vi "RealSense_HelloWorld_PointCloud.vi"() -> ()   [LabVIEW 2017]
doc: "Simple Demo showing how to connect a RealSense Camera to stream COLOR and DEPTH from the stereo camera of a D4xx series camera."
uses:
  <vilib>/Utility/miscctls.llb/LV3DPointTypeDef.ctl
  <vilib>/Utility/miscctls.llb/LVRGBAColorTypeDef.ctl
  <vilib>/picture/3D Picture Control/Object/Create Object (name).vi
  libRealSense3.lvlib
  <vilib>/picture/3D Picture Control/NI_3D Picture Control.lvlib
panel:
  in  "Color format":enum16{"Monochrome", "RGB internal (RGB)"}(ring)=enum."RGB internal (RGB)"
  in  "Display tab":T1(tab)
  out "Stream selection":u16(ring) items=["Depth + Left Color", "Unrectified L + R", "Rectified L + R", "Depth Only", "RGB ext. Only", "Depth + L Monochrome"]
  out "Found \nRealSense":bool=TRUE
  out "height":i32=720
  out "width":i32=1280
  out "init results":T2={"camera name"="Intel RealSense D415", "camera S/N"="725112060291", "F/W"="05.12.01.00", "Sensor name"="Stereo Module", "api_version"=23201, "rscontext"=2279652045952, "device_list"=2279390748064, "device count"=1, "Dev out"=2279652602464, "sensor_list"=2279759543328, "sensor count"=2, "Sensor out"=2279397784752}
  in  "Select Resolution":u16(ring)=29 items=["256 x 144 @90fps", "424 x 240 @6fps", "424 x 240 @15fps", "424 x 240 @30fps", "424 x 240 @60fps", "424 x 240 @90fps", "480 x 270 @6fps", "480 x 270 @15fps", "480 x 270 @30fps", "480 x 270 @60fps", "480 x 270 @90fps", "640 x 360 @6fps", "640 x 360 @15fps", "640 x 360 @30fps", "640 x 360 @60fps", "640 x 360 @90fps", "640 x 480 @6fps", "640 x 480 @15fps", "640 x 480 @30fps", "640 x 480 @60fps", "640 x 480 @90fps", "848 x 100 @100fps", "848 x 480 @6fps", "848 x 480 @15fps", "848 x 480 @30fps", "848 x 480 @60fps", "848 x 480 @90fps", "1280 x 720 @6fps", "1280 x 720 @15fps", "1280 x 720 @30fps"]
  in  "Sensor index":i32
  in  "Device index":i32
  out "L-R Baseline, mm":sgl=-54.83181
  out "fy":sgl=952.6064 format="%#_5g"
  out "fx":sgl=952.6064 format="%#_5g"
  out "ppy":sgl=370.69974 format="%#_5g"
  out "ppx":sgl=634.5728 format="%#_5g"
  in  "Exposure,us":sgl=33000.0
  in  "Autoexposure":bool=TRUE
  in  "Depth Presets":T3(ring)=enum."Face2"
  in  "Color Presets":T4(ring)=enum."DS410 (DS5a) 4"
  in  "Laser on/off":bool=TRUE
  in  "Gain(16-248)":sgl=16.0 min=16 max=248
  in  "Update Presets":bool
  in  "Laser \nPower (mW)":dbl(slide)=155.72448 min=0.0 max=360.0 scale=0.36..360.0
  in  "Range Scale":enum16{"200m", "100m", "60m", "6m", "2m", "1m"}(ring)=enum."6m"
  out "RGB image":picture
  out "Depth map":sgl[][](graph)
  out "3D Picture":refnum<vi>(3d-picture)
  out "init error":string="\rNo Error\rNo Error\rNo Error\rNo Error\rNo Error\rNo Error\rNo Error\r\rNo Error\rNo Error"
  out "Capture2 error":string="No Error"
  out "Start Error":string="No Error\rNo Error\rNo Error"
  out "Config error":string="No Error\rNo Error"
  out "Capture1 Error":string="No Error"
  out "Close Error":string="No Error\rNo Error\rNo Error\rNo Error"
  out "release frame error":string="No Error"
  out "iteration":i32=187
  in  "stop":bool=TRUE
  # "RealSense Hello World: PointCloud"
  # "This demo shows how to connect a RealSense D415 (not 435) Depth Camera, and display the textured PointCloud."
  # "Note; When you change Depth Preset you need to stop and restart for the HDAD settings to take effect.\n\nTry the Color preset called \"Remove IR2\". It will remove the laser projector from the RGB 1280x720 image."
  # "INTRINSICS & EXTRINSICS"
  # "SELECT THE RESOLUTION"
  # "Recommendation:\nFor D435: 848x480, D415: 1280x720"
  # "DEPTH MAP"
  # "COLOR"
  # "Changes Color scale for Depth Map."
  # "20-1660000"
  # "3D POINTCLOUD"
  # "Rotate: Drag image\nMove X-Y: HOLD DOWN CTRL while dragging.\nZoom: SHIFT while dragging."
  # "ERRORS"
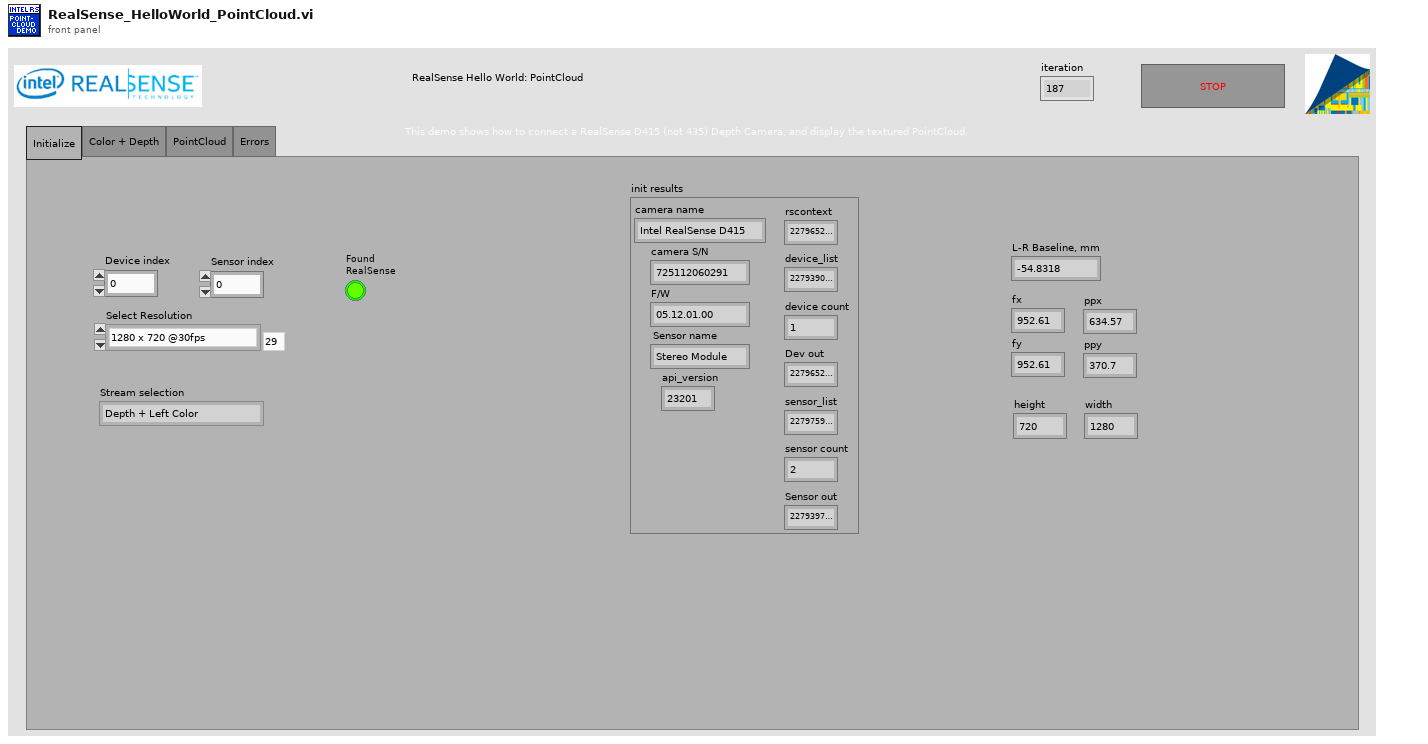
[diagram p1: front panel]
types:
  T1 = enum32{"Initialize", "Color + Depth", "PointCloud", "Errors"}
  T2 = cluster{"camera name":string, "camera S/N":string, "F/W":string, "Sensor name":string, "api_version":i32, "rscontext":u64, "device_list":u64, "device count":i32, "Dev out":u64, "sensor_list":u64, "sensor count":i32, "Sensor out":u64}
  T3 = enum16{"Custom", "Original", "New Depth 1", "New Depth 2", "Depth Active 1", "Active 3D Scan", "Active Short A", "Active Short C", "Face", "Face2", "Best Box", "High Density", "Medium Density", "High Accuracy", "Hand", "Short Range", "Flat wall", "Load .JSON", "Load .JSON2"}
  T4 = enum16{"Custom", "RS400 (DS5p)", "RS400 (DS5p) 2", "RS400 (DS5p) 3", "RS400 (DS5p) 4", "RS400 (DS5p) 5", "RS410 (DS5a)", "RS410 (DS5a) 2", "DS410 (DS5a) 3", "DS410 (DS5a) 4", "DS410+IR", "DS5LR", "DS5LR-2", "DS5LR no pattern", "RS410 Remove IR", "RS410 Remove IR 2", "DS5micro", "D435"}
  T5 = cluster{"width":i32, "height":i32, "fps":i32, "Profile":u64, "ppx":sgl, "ppy":sgl, "fx":sgl, "fy":sgl, "model":u32}
  T6 = enum16{"Overall", "Per Primitive", "Per Vertex", "Binding Off"}
  T7 = enum16{"Points", "Lines", "Line Strip", "Line Loop", "Triangles", "Triangle Strip", "Triangle Fan", "Quads", "Quad Strip", "Polygon"}
  T8 = enum16{"Depth", "Color (ext.)", "Color (left) ", "IR Left", "IR Right", "IR Left (Y16)", "IR Right (Y16)"}
  T9 = cluster{"R":dbl, "G":dbl, "B":dbl, "Alpha":dbl}[]
  T10 = typedef "LVRGBAColorTypeDef.ctl" = cluster{"Red":sgl, "Green":sgl, "Blue":sgl, "Alpha":sgl}
  T11 = typedef "LV3DPointTypeDef.ctl" = cluster{"X":sgl, "Y":sgl, "Z":sgl}
  T12 = cluster{"Alpha":sgl, "Blue":sgl, "Green":sgl, "Red":sgl}
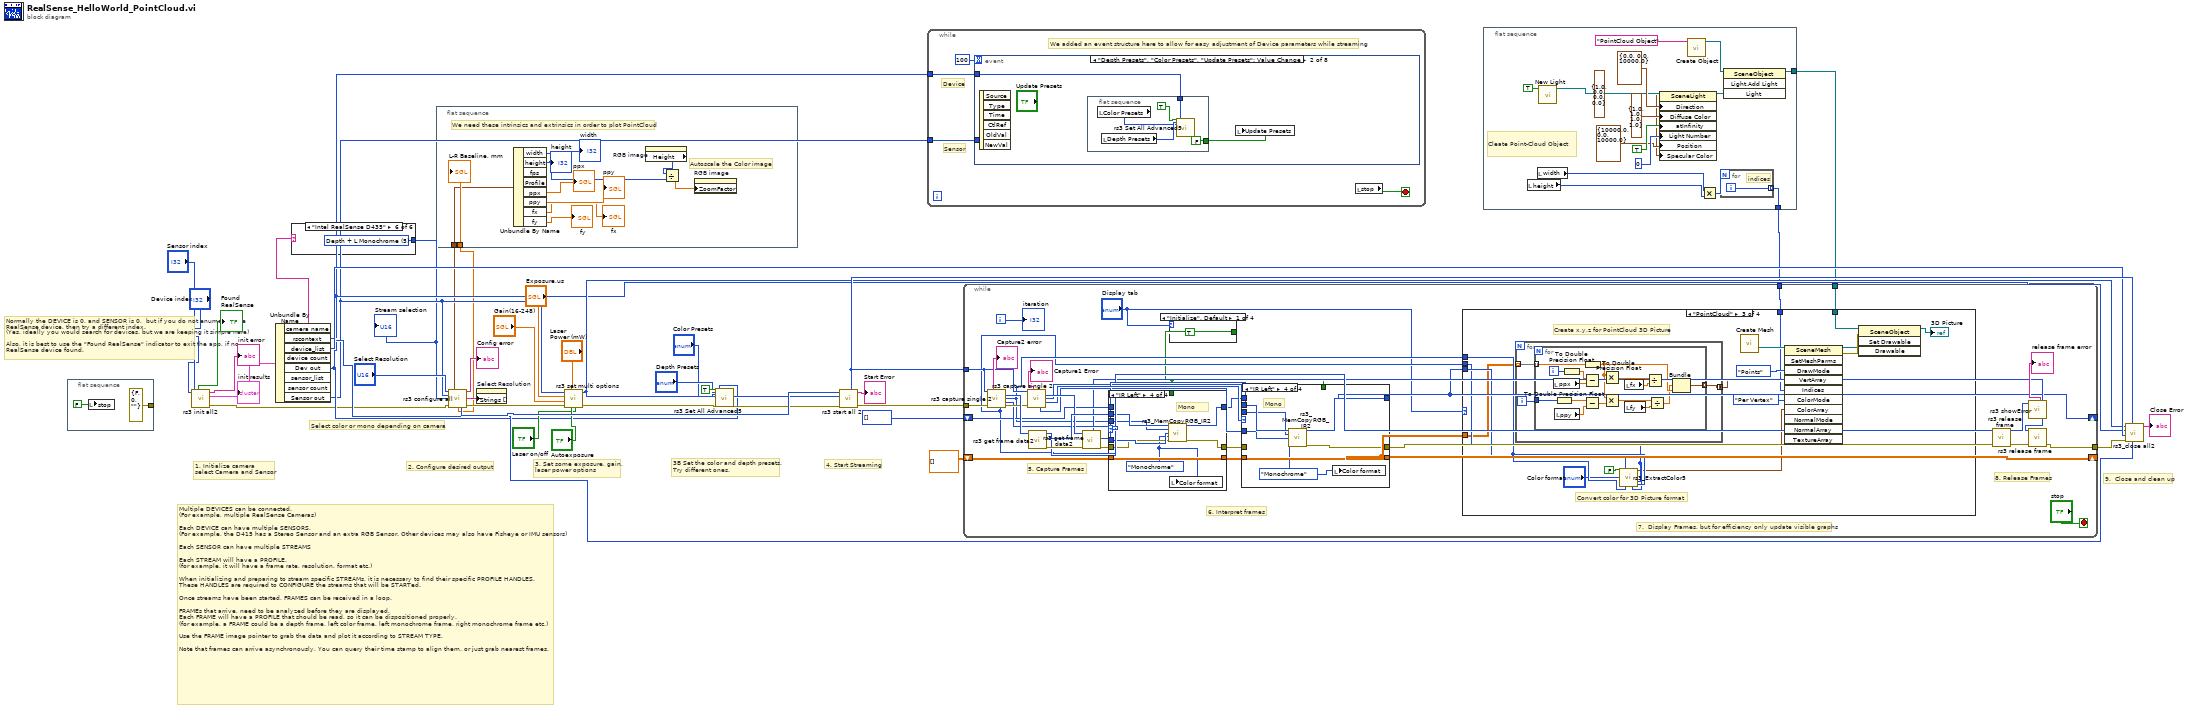
[diagram p0: block diagram]
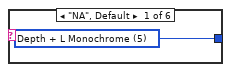
[diagram p2: hidden frame]
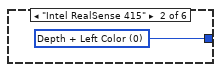
[diagram p3: hidden frame]
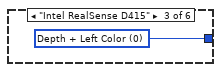
[diagram p4: hidden frame]
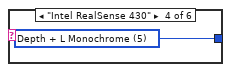
[diagram p5: hidden frame]
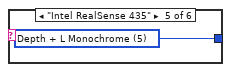
[diagram p6: hidden frame]
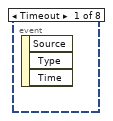
[diagram p7: hidden frame]
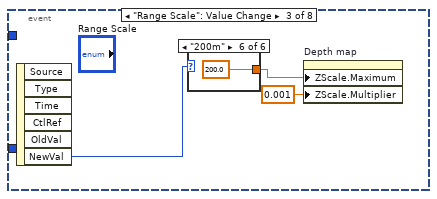
[diagram p8: hidden frame]
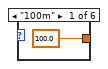
[diagram p9: hidden frame]
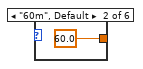
[diagram p10: hidden frame]
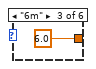
[diagram p11: hidden frame]
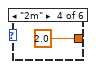
[diagram p12: hidden frame]
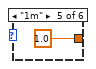
[diagram p13: hidden frame]
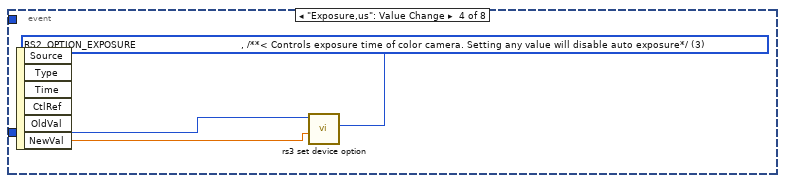
[diagram p14: hidden frame]
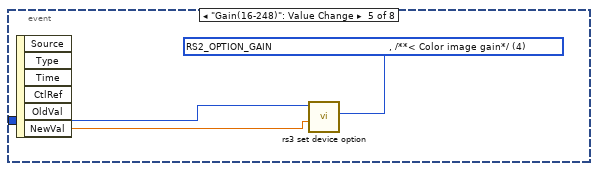
[diagram p15: hidden frame]
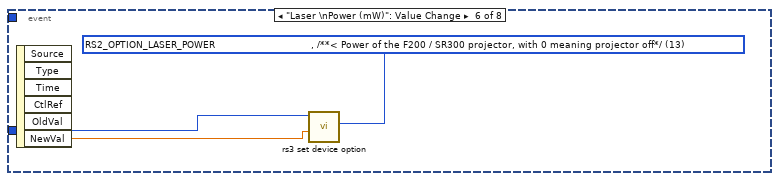
[diagram p16: hidden frame]
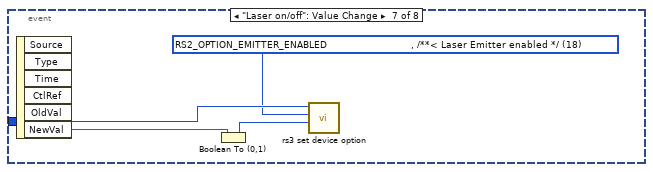
[diagram p17: hidden frame]
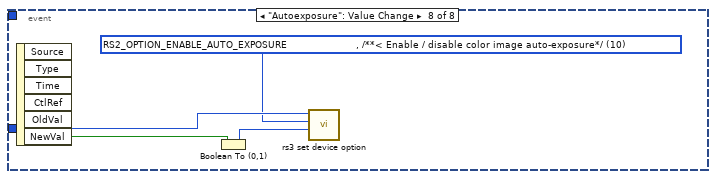
[diagram p18: hidden frame]
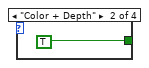
[diagram p19: hidden frame]
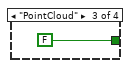
[diagram p20: hidden frame]
diagram:
  # "3B Set the color and depth presets.\nTry different ones."
  # "Select color or mono depending on camera"
  # "Normally the DEVICE is 0, and SENSOR is 0,  but if you do not enumerate the RealSense device, then try a different index.\n(Yes, ideally you would search for devices, but we are keeping it simple here)\n\nAlso, it is best to use the \"Found RealSense\" indicator to exit the app, if no RealSense device found."
  # "Multiple DEVICES can be connected. \n(For example, multiple RealSense Cameras)\n\nEach DEVICE can have multiple SENSORS. \n(For example, the D415 has a Stereo Sensor and an extra RGB Sensor. Other devices may also have Fisheye or IMU sensors) \n\nEach SENSOR can have multiple STREAMS\n\nEach STREAM will have a PROFILE. \n(for example, it will have a frame rate, resolution, format etc.)\n\nWhen initializing and preparing to stream specific STREAMs, it is necessary to find their specific PROFILE HANDLES.\nThese HANDLES are required to CONFIGURE the streams that will be STARTed. \n\nOnce streams have been started, FRAMES can be received in a loop. \n \nFRAMEs that arrive, need to be analyzed before they are displayed. \nEach FRAME will have a PROFILE that should be read, so it can be dispositioned properly.\n(for example, a FRAME could be a depth frame, left color frame, left monochrome frame, right monochrome frame etc.)\n\nUse the FRAME image pointer to grab the data and plot it according to STREAM TYPE.\n\nNote that frames can arrive asynchronously. You can query their time stamp to align them, or just grab nearest frames."
  # "9.  Close and clean up"
  # "4. Start Streaming"
  # "3. Set some exposure, gain, \nlaser power options"
  # "2. Configure desired output"
  # "1. Initialize camera\nselect Camera and Sensor"
  n1 = flat-sequence {
    tunnel: [errorcluster {"status"=FALSE, "code"=0, "source"=""} ("error in")] -> _
    frame #0 {
      n2 = local write "stop"(FALSE ("stop")) -> ()
    }
  }
  n3 = call "rs3 init all2.vi"("Select Device"="Device index", "Select Sensor"="Sensor index") -> ("error out"=w3:errorcluster, "init results"=w8:T2, "init error"=→"init error":string, "Found RealSense"=→"Found \nRealSense":bool)  [unwired: 3 in, 3 out]
  "init results" <- w8
  n4 = Unbundle By Name(w8) -> ("camera name"=w2:string, "rscontext"=w33:u64, "device_list"=w34:u64, "Dev out"=w16:u64, "Sensor out"=w15:u64)  [unwired: 3 out]
  n5 = case shown="\"Intel RealSense D435\"" w2 {
    tunnel: [w42 w43 w44 w45 w46 w47] -> w1
    frame "NA", Default {
      w42 = u16 5 items=["Depth + Left Color", "Unrectified L + R", "Rectified L + R", "Depth Only", "RGB ext. Only", "Depth + L Monochrome"] ("Stream selection")
    }
    frame "Intel RealSense 415" {
      w43 = u16 0 items=["Depth + Left Color", "Unrectified L + R", "Rectified L + R", "Depth Only", "RGB ext. Only", "Depth + L Monochrome"] ("Stream selection")
    }
    frame "Intel RealSense D415" {
      w44 = u16 0 items=["Depth + Left Color", "Unrectified L + R", "Rectified L + R", "Depth Only", "RGB ext. Only", "Depth + L Monochrome"] ("Stream selection")
    }
    frame "Intel RealSense 430" {
      w45 = u16 5 items=["Depth + Left Color", "Unrectified L + R", "Rectified L + R", "Depth Only", "RGB ext. Only", "Depth + L Monochrome"] ("Stream selection")
    }
    frame "Intel RealSense 435" {
      w46 = u16 5 items=["Depth + Left Color", "Unrectified L + R", "Rectified L + R", "Depth Only", "RGB ext. Only", "Depth + L Monochrome"] ("Stream selection")
    }
    frame "Intel RealSense D435" {
      w47 = u16 5 items=["Depth + Left Color", "Unrectified L + R", "Rectified L + R", "Depth Only", "RGB ext. Only", "Depth + L Monochrome"] ("Stream selection")
    }
  }
  "Stream selection" <- w1
  n6 = flat-sequence {
    tunnel: w13 -> [w57]
    tunnel: w12 -> [w56]
    frame #0 {
      # "Autoscale the Color image"
      # "We need these intrinsics and extrinsics in order to plot PointCloud"
      n7 = Unbundle By Name(w56) -> ("width"=→"width":i32, "height"=w54:i32, "ppx"=→"ppx":sgl, "ppy"=→"ppy":sgl, "fx"=→"fx":sgl, "fy"=→"fy":sgl)  [unwired: 2 out]
      "height" <- w54
      n8 = property on="RGB image" class="Pict"() -> ("Height"=w55:u32)  [unwired: 2 in, 2 out]
      n9 = Divide(x=w55, y=w54) -> (x/y=w53:dbl)
      n10 = property on="RGB image" class="Pict"("ZoomFactor"=w53) -> ()  [unwired: 2 in, 2 out]
      "L-R Baseline, mm" <- w57
    }
  }
  n11 = call "rs3 configure all.vi"("Select Resolution"="Select Resolution", "Sensor in"=w15, "Stream selection"=w1, "error in (no error)"=w3) -> ("Output stream L"=w12:T5, "config error"=→"Config error":string, "Output stream"=w29:string[], "L-R Baseline, mm"=w13:sgl, "Stream Profile Handles"=w39:u64[], "error out"=w28:errorcluster)  [unwired: 2 in, 4 out]
  n12 = property on="Select Resolution" class="Ring (strict)"("Strings []"=w29) -> ()  [unwired: 2 in, 2 out]
  n13 = call "rs3 set multi options.vi"("laser on/off"="Laser on/off", "autoexposure"="Autoexposure", "Laser power, mW (0-360)"="Laser \nPower (mW)", "error in (no error)"=w28, "Gain(16-248)"="Gain(16-248)", "Exposure, us"="Exposure,us", "Sensor in"=w15) -> ("error out"=w21:errorcluster, "Sensor out"=w27:u64)  [unwired: 2 in, 1 out]
  n14 = call "rs3 Set All Advanced5.vi"("Set Color Corr"=TRUE, "Depth Presets"="Depth Presets", "Color Presets"="Color Presets", "error in (no error)"=w21, "device in"=w16) -> ("error out"=w20:errorcluster)  [unwired: 20 in, 2 out]
  n15 = call "rs3 start all 2.vi"("error in (no error)"=w20, "Sensor in"=w27, "Stream profile array"=w39) -> ("error out"=w30:errorcluster, "Config Error"=→"Start Error":string, "queue out"=w38:u64)  [unwired: 5 in, 1 out]
  n16 = while {
    tunnel: w16 -> [w60]
    tunnel: w15 -> [w59]
    stop <- w61 stop-if-true
    # "Sensor"
    # "Device"
    # "We added an event structure here to allow for easy adjustment of Device parameters while streaming"
    n17 = event shown="[1] \"Depth Presets\", \"Color Presets\", \"Update Presets\": Value Change" {
      selector: _ -> [_ _ _ _ _ _ _ _]
      dyn-events: _ -> [_ _ _ _ _ _ _ _]
      timeout: 100 -> [_ _ _ _ _ _ _ _]
      tunnel: w60 -> [_ w63 _ _ _ _ _ _]
      tunnel: w59 -> [_ _ _ w80 w83 w86 w90 w94]
      event Timeout {
        n18 = event-data() -> ()  [unwired: 1 in, 3 out]
      }
      event "Depth Presets", "Color Presets", "Update Presets": Value Change {
        n19 = event-data() -> ()  [unwired: 1 in, 6 out]
        n20 = flat-sequence {
          tunnel: w63 -> [w65]
          tunnel: [FALSE ("Update Presets")] -> w62
          frame #0 {
            n21 = local read "Color Presets"() -> (w67:T4)
            n22 = local read "Depth Presets"() -> (w68:T3)
            n23 = call "rs3 Set All Advanced5.vi"("Set Color Corr"=TRUE, "Depth Presets"=w68, "Color Presets"=w67, "device in"=w65) -> ()  [unwired: 21 in, 3 out]
          }
        }
        n24 = local write "Update Presets"(w62) -> ()
      }
      event "Range Scale": Value Change {
        n25 = event-data() -> ("NewVal"=w70:enum16{"200m", "100m", "60m", "6m", "2m", "1m"})  [unwired: 1 in, 5 out]
        n26 = case shown="\"200m\"" w70 {
          tunnel: [100.0 ("Z Scale.Offset and Multiplier:Multiplier") 60.0 ("Z Scale.Offset and Multiplier:Multiplier") 6.0 ("Z Scale.Offset and Multiplier:Multiplier") 2.0 ("Z Scale.Offset and Multiplier:Multiplier") 1.0 ("Z Scale.Offset and Multiplier:Multiplier") 200.0 ("Z Scale.Offset and Multiplier:Multiplier")] -> w69
          frame "100m" {
          }
          frame "60m", Default {
          }
          frame "6m" {
          }
          frame "2m" {
          }
          frame "1m" {
          }
          frame "200m" {
          }
        }
        n27 = property on="Depth map" class="IntGraph (strict)"("ZScale.Maximum"=w69, "ZScale.Multiplier"=0.001 ("Z Scale.Offset and Multiplier:Multiplier")) -> ()  [unwired: 2 in, 2 out]
      }
      event "Exposure,us": Value Change {
        w78 = u16 3 items=["    RS2_OPTION_BACKLIGHT_COMPENSATION                     , /**< Enable / disable color backlight compensation*/", "    RS2_OPTION_BRIGHTNESS                                 , /**< Color image brightness*/", "    RS2_OPTION_CONTRAST                                   , /**< Color image contrast*/", "    RS2_OPTION_EXPOSURE                                   , /**< Controls exposure time of color camera. Setting any value will disable auto exposure*/", "    RS2_OPTION_GAIN                                       , /**< Color image gain*/", "    RS2_OPTION_GAMMA                                      , /**< Color image gamma setting*/", "    RS2_OPTION_HUE                                        , /**< Color image hue*/", "    RS2_OPTION_SATURATION                                 , /**< Color image saturation setting*/", "    RS2_OPTION_SHARPNESS                                  , /**< Color image sharpness setting*/", "    RS2_OPTION_WHITE_BALANCE                              , /**< Controls white balance of color image. Setting any value will disable auto white balance*/", "    RS2_OPTION_ENABLE_AUTO_EXPOSURE                       , /**< Enable / disable color image auto-exposure*/", "    RS2_OPTION_ENABLE_AUTO_WHITE_BALANCE                  , /**< Enable / disable color image auto-white-balance*/", "    RS2_OPTION_VISUAL_PRESET                              , /**< Provide access to several recommend sets of option presets for the depth camera */", "    RS2_OPTION_LASER_POWER                                , /**< Power of the F200 / SR300 projector, with 0 meaning projector off*/", "    RS2_OPTION_ACCURACY                                   , /**< Set the number of patterns projected per frame. The higher the accuracy value the more patterns projected. Increasing the number of patterns help to achieve better accuracy. Note that this c", "    RS2_OPTION_MOTION_RANGE                               , /**< Motion vs. Range trade-off, with lower values allowing for better motion sensitivity and higher values allowing for better depth range*/", "    RS2_OPTION_FILTER_OPTION                              , /**< Set the filter to apply to each depth frame. Each one of the filter is optimized per the application requirements*/", "    RS2_OPTION_CONFIDENCE_THRESHOLD                       , /**< The confidence level threshold used by the Depth algorithm pipe to set whether a pixel will get a valid range or will be marked with invalid range*/", "    RS2_OPTION_EMITTER_ENABLED                            , /**< Laser Emitter enabled */", "    RS2_OPTION_FRAMES_QUEUE_SIZE                          , /**< Number of frames the user is allowed to keep per stream. Trying to hold-on to more frames will cause frame-drops.*/", "    RS2_OPTION_TOTAL_FRAME_DROPS                          , /**< Total number of detected frame drops from all streams */", "    RS2_OPTION_AUTO_EXPOSURE_MODE                         , /**< Auto-Exposure modes: Static, Anti-Flicker and Hybrid */", "    RS2_OPTION_POWER_LINE_FREQUENCY                       , /**< Power Line Frequency control for anti-flickering Off/50Hz/60Hz/Auto */", "    RS2_OPTION_ASIC_TEMPERATURE                           , /**< Current Asic Temperature */", "    RS2_OPTION_ERROR_POLLING_ENABLED                      , /**< disable error handling */", "    RS2_OPTION_PROJECTOR_TEMPERATURE                      , /**< Current Projector Temperature */", "    RS2_OPTION_OUTPUT_TRIGGER_ENABLED                     , /**< Enable / disable trigger to be outputed from the camera to any external device on every depth frame */", "    RS2_OPTION_MOTION_MODULE_TEMPERATURE                  , /**< Current Motion-Module Temperature */", "    RS2_OPTION_DEPTH_UNITS                                , /**< Number of meters represented by a single depth unit */", "    RS2_OPTION_ENABLE_MOTION_CORRECTION                   , /**< Enable/Disable automatic correction of the motion data */", "    RS2_OPTION_AUTO_EXPOSURE_PRIORITY                     , /**< Allows sensor to dynamically ajust the frame rate depending on lighting conditions */", "    RS2_OPTION_COUNT                                      , /**< Number of enumeration values. Not a valid input: intended to be used in for-loops. */"] ("RS Option")
        n28 = event-data() -> ("NewVal"=w79:sgl)  [unwired: 1 in, 5 out]
        n29 = call "rs3 set device option.vi"("value"=w79, "RS Option"=w78, "Sensor in"=w80) -> ()  [unwired: 6 in, 3 out]
      }
      event "Gain(16-248)": Value Change {
        w81 = u16 4 items=["    RS2_OPTION_BACKLIGHT_COMPENSATION                     , /**< Enable / disable color backlight compensation*/", "    RS2_OPTION_BRIGHTNESS                                 , /**< Color image brightness*/", "    RS2_OPTION_CONTRAST                                   , /**< Color image contrast*/", "    RS2_OPTION_EXPOSURE                                   , /**< Controls exposure time of color camera. Setting any value will disable auto exposure*/", "    RS2_OPTION_GAIN                                       , /**< Color image gain*/", "    RS2_OPTION_GAMMA                                      , /**< Color image gamma setting*/", "    RS2_OPTION_HUE                                        , /**< Color image hue*/", "    RS2_OPTION_SATURATION                                 , /**< Color image saturation setting*/", "    RS2_OPTION_SHARPNESS                                  , /**< Color image sharpness setting*/", "    RS2_OPTION_WHITE_BALANCE                              , /**< Controls white balance of color image. Setting any value will disable auto white balance*/", "    RS2_OPTION_ENABLE_AUTO_EXPOSURE                       , /**< Enable / disable color image auto-exposure*/", "    RS2_OPTION_ENABLE_AUTO_WHITE_BALANCE                  , /**< Enable / disable color image auto-white-balance*/", "    RS2_OPTION_VISUAL_PRESET                              , /**< Provide access to several recommend sets of option presets for the depth camera */", "    RS2_OPTION_LASER_POWER                                , /**< Power of the F200 / SR300 projector, with 0 meaning projector off*/", "    RS2_OPTION_ACCURACY                                   , /**< Set the number of patterns projected per frame. The higher the accuracy value the more patterns projected. Increasing the number of patterns help to achieve better accuracy. Note that this c", "    RS2_OPTION_MOTION_RANGE                               , /**< Motion vs. Range trade-off, with lower values allowing for better motion sensitivity and higher values allowing for better depth range*/", "    RS2_OPTION_FILTER_OPTION                              , /**< Set the filter to apply to each depth frame. Each one of the filter is optimized per the application requirements*/", "    RS2_OPTION_CONFIDENCE_THRESHOLD                       , /**< The confidence level threshold used by the Depth algorithm pipe to set whether a pixel will get a valid range or will be marked with invalid range*/", "    RS2_OPTION_EMITTER_ENABLED                            , /**< Laser Emitter enabled */", "    RS2_OPTION_FRAMES_QUEUE_SIZE                          , /**< Number of frames the user is allowed to keep per stream. Trying to hold-on to more frames will cause frame-drops.*/", "    RS2_OPTION_TOTAL_FRAME_DROPS                          , /**< Total number of detected frame drops from all streams */", "    RS2_OPTION_AUTO_EXPOSURE_MODE                         , /**< Auto-Exposure modes: Static, Anti-Flicker and Hybrid */", "    RS2_OPTION_POWER_LINE_FREQUENCY                       , /**< Power Line Frequency control for anti-flickering Off/50Hz/60Hz/Auto */", "    RS2_OPTION_ASIC_TEMPERATURE                           , /**< Current Asic Temperature */", "    RS2_OPTION_ERROR_POLLING_ENABLED                      , /**< disable error handling */", "    RS2_OPTION_PROJECTOR_TEMPERATURE                      , /**< Current Projector Temperature */", "    RS2_OPTION_OUTPUT_TRIGGER_ENABLED                     , /**< Enable / disable trigger to be outputed from the camera to any external device on every depth frame */", "    RS2_OPTION_MOTION_MODULE_TEMPERATURE                  , /**< Current Motion-Module Temperature */", "    RS2_OPTION_DEPTH_UNITS                                , /**< Number of meters represented by a single depth unit */", "    RS2_OPTION_ENABLE_MOTION_CORRECTION                   , /**< Enable/Disable automatic correction of the motion data */", "    RS2_OPTION_AUTO_EXPOSURE_PRIORITY                     , /**< Allows sensor to dynamically ajust the frame rate depending on lighting conditions */", "    RS2_OPTION_COUNT                                      , /**< Number of enumeration values. Not a valid input: intended to be used in for-loops. */"] ("RS Option")
        n30 = event-data() -> ("NewVal"=w82:sgl)  [unwired: 1 in, 5 out]
        n31 = call "rs3 set device option.vi"("value"=w82, "RS Option"=w81, "Sensor in"=w83) -> ()  [unwired: 6 in, 3 out]
      }
      event "Laser \nPower (mW)": Value Change {
        w84 = u16 13 items=["    RS2_OPTION_BACKLIGHT_COMPENSATION                     , /**< Enable / disable color backlight compensation*/", "    RS2_OPTION_BRIGHTNESS                                 , /**< Color image brightness*/", "    RS2_OPTION_CONTRAST                                   , /**< Color image contrast*/", "    RS2_OPTION_EXPOSURE                                   , /**< Controls exposure time of color camera. Setting any value will disable auto exposure*/", "    RS2_OPTION_GAIN                                       , /**< Color image gain*/", "    RS2_OPTION_GAMMA                                      , /**< Color image gamma setting*/", "    RS2_OPTION_HUE                                        , /**< Color image hue*/", "    RS2_OPTION_SATURATION                                 , /**< Color image saturation setting*/", "    RS2_OPTION_SHARPNESS                                  , /**< Color image sharpness setting*/", "    RS2_OPTION_WHITE_BALANCE                              , /**< Controls white balance of color image. Setting any value will disable auto white balance*/", "    RS2_OPTION_ENABLE_AUTO_EXPOSURE                       , /**< Enable / disable color image auto-exposure*/", "    RS2_OPTION_ENABLE_AUTO_WHITE_BALANCE                  , /**< Enable / disable color image auto-white-balance*/", "    RS2_OPTION_VISUAL_PRESET                              , /**< Provide access to several recommend sets of option presets for the depth camera */", "    RS2_OPTION_LASER_POWER                                , /**< Power of the F200 / SR300 projector, with 0 meaning projector off*/", "    RS2_OPTION_ACCURACY                                   , /**< Set the number of patterns projected per frame. The higher the accuracy value the more patterns projected. Increasing the number of patterns help to achieve better accuracy. Note that this c", "    RS2_OPTION_MOTION_RANGE                               , /**< Motion vs. Range trade-off, with lower values allowing for better motion sensitivity and higher values allowing for better depth range*/", "    RS2_OPTION_FILTER_OPTION                              , /**< Set the filter to apply to each depth frame. Each one of the filter is optimized per the application requirements*/", "    RS2_OPTION_CONFIDENCE_THRESHOLD                       , /**< The confidence level threshold used by the Depth algorithm pipe to set whether a pixel will get a valid range or will be marked with invalid range*/", "    RS2_OPTION_EMITTER_ENABLED                            , /**< Laser Emitter enabled */", "    RS2_OPTION_FRAMES_QUEUE_SIZE                          , /**< Number of frames the user is allowed to keep per stream. Trying to hold-on to more frames will cause frame-drops.*/", "    RS2_OPTION_TOTAL_FRAME_DROPS                          , /**< Total number of detected frame drops from all streams */", "    RS2_OPTION_AUTO_EXPOSURE_MODE                         , /**< Auto-Exposure modes: Static, Anti-Flicker and Hybrid */", "    RS2_OPTION_POWER_LINE_FREQUENCY                       , /**< Power Line Frequency control for anti-flickering Off/50Hz/60Hz/Auto */", "    RS2_OPTION_ASIC_TEMPERATURE                           , /**< Current Asic Temperature */", "    RS2_OPTION_ERROR_POLLING_ENABLED                      , /**< disable error handling */", "    RS2_OPTION_PROJECTOR_TEMPERATURE                      , /**< Current Projector Temperature */", "    RS2_OPTION_OUTPUT_TRIGGER_ENABLED                     , /**< Enable / disable trigger to be outputed from the camera to any external device on every depth frame */", "    RS2_OPTION_MOTION_MODULE_TEMPERATURE                  , /**< Current Motion-Module Temperature */", "    RS2_OPTION_DEPTH_UNITS                                , /**< Number of meters represented by a single depth unit */", "    RS2_OPTION_ENABLE_MOTION_CORRECTION                   , /**< Enable/Disable automatic correction of the motion data */", "    RS2_OPTION_AUTO_EXPOSURE_PRIORITY                     , /**< Allows sensor to dynamically ajust the frame rate depending on lighting conditions */", "    RS2_OPTION_COUNT                                      , /**< Number of enumeration values. Not a valid input: intended to be used in for-loops. */"] ("RS Option")
        n32 = event-data() -> ("NewVal"=w85:dbl)  [unwired: 1 in, 5 out]
        n33 = call "rs3 set device option.vi"("value"=w85, "RS Option"=w84, "Sensor in"=w86) -> ()  [unwired: 6 in, 3 out]
      }
      event "Laser on/off": Value Change {
        w89 = u16 18 items=["    RS2_OPTION_BACKLIGHT_COMPENSATION                     , /**< Enable / disable color backlight compensation*/", "    RS2_OPTION_BRIGHTNESS                                 , /**< Color image brightness*/", "    RS2_OPTION_CONTRAST                                   , /**< Color image contrast*/", "    RS2_OPTION_EXPOSURE                                   , /**< Controls exposure time of color camera. Setting any value will disable auto exposure*/", "    RS2_OPTION_GAIN                                       , /**< Color image gain*/", "    RS2_OPTION_GAMMA                                      , /**< Color image gamma setting*/", "    RS2_OPTION_HUE                                        , /**< Color image hue*/", "    RS2_OPTION_SATURATION                                 , /**< Color image saturation setting*/", "    RS2_OPTION_SHARPNESS                                  , /**< Color image sharpness setting*/", "    RS2_OPTION_WHITE_BALANCE                              , /**< Controls white balance of color image. Setting any value will disable auto white balance*/", "    RS2_OPTION_ENABLE_AUTO_EXPOSURE                       , /**< Enable / disable color image auto-exposure*/", "    RS2_OPTION_ENABLE_AUTO_WHITE_BALANCE                  , /**< Enable / disable color image auto-white-balance*/", "    RS2_OPTION_VISUAL_PRESET                              , /**< Provide access to several recommend sets of option presets for the depth camera */", "    RS2_OPTION_LASER_POWER                                , /**< Power of the F200 / SR300 projector, with 0 meaning projector off*/", "    RS2_OPTION_ACCURACY                                   , /**< Set the number of patterns projected per frame. The higher the accuracy value the more patterns projected. Increasing the number of patterns help to achieve better accuracy. Note that this c", "    RS2_OPTION_MOTION_RANGE                               , /**< Motion vs. Range trade-off, with lower values allowing for better motion sensitivity and higher values allowing for better depth range*/", "    RS2_OPTION_FILTER_OPTION                              , /**< Set the filter to apply to each depth frame. Each one of the filter is optimized per the application requirements*/", "    RS2_OPTION_CONFIDENCE_THRESHOLD                       , /**< The confidence level threshold used by the Depth algorithm pipe to set whether a pixel will get a valid range or will be marked with invalid range*/", "    RS2_OPTION_EMITTER_ENABLED                            , /**< Laser Emitter enabled */", "    RS2_OPTION_FRAMES_QUEUE_SIZE                          , /**< Number of frames the user is allowed to keep per stream. Trying to hold-on to more frames will cause frame-drops.*/", "    RS2_OPTION_TOTAL_FRAME_DROPS                          , /**< Total number of detected frame drops from all streams */", "    RS2_OPTION_AUTO_EXPOSURE_MODE                         , /**< Auto-Exposure modes: Static, Anti-Flicker and Hybrid */", "    RS2_OPTION_POWER_LINE_FREQUENCY                       , /**< Power Line Frequency control for anti-flickering Off/50Hz/60Hz/Auto */", "    RS2_OPTION_ASIC_TEMPERATURE                           , /**< Current Asic Temperature */", "    RS2_OPTION_ERROR_POLLING_ENABLED                      , /**< disable error handling */", "    RS2_OPTION_PROJECTOR_TEMPERATURE                      , /**< Current Projector Temperature */", "    RS2_OPTION_OUTPUT_TRIGGER_ENABLED                     , /**< Enable / disable trigger to be outputed from the camera to any external device on every depth frame */", "    RS2_OPTION_MOTION_MODULE_TEMPERATURE                  , /**< Current Motion-Module Temperature */", "    RS2_OPTION_DEPTH_UNITS                                , /**< Number of meters represented by a single depth unit */", "    RS2_OPTION_ENABLE_MOTION_CORRECTION                   , /**< Enable/Disable automatic correction of the motion data */", "    RS2_OPTION_AUTO_EXPOSURE_PRIORITY                     , /**< Allows sensor to dynamically ajust the frame rate depending on lighting conditions */", "    RS2_OPTION_COUNT                                      , /**< Number of enumeration values. Not a valid input: intended to be used in for-loops. */"] ("RS Option")
        n34 = event-data() -> ("NewVal"=w88:bool)  [unwired: 1 in, 5 out]
        n35 = Boolean To (0,1)(Boolean=w88) -> (0, 1=w87:i16)
        n36 = call "rs3 set device option.vi"("value"=w87, "RS Option"=w89, "Sensor in"=w90) -> ()  [unwired: 6 in, 3 out]
      }
      event "Autoexposure": Value Change {
        w93 = u16 10 items=["    RS2_OPTION_BACKLIGHT_COMPENSATION                     , /**< Enable / disable color backlight compensation*/", "    RS2_OPTION_BRIGHTNESS                                 , /**< Color image brightness*/", "    RS2_OPTION_CONTRAST                                   , /**< Color image contrast*/", "    RS2_OPTION_EXPOSURE                                   , /**< Controls exposure time of color camera. Setting any value will disable auto exposure*/", "    RS2_OPTION_GAIN                                       , /**< Color image gain*/", "    RS2_OPTION_GAMMA                                      , /**< Color image gamma setting*/", "    RS2_OPTION_HUE                                        , /**< Color image hue*/", "    RS2_OPTION_SATURATION                                 , /**< Color image saturation setting*/", "    RS2_OPTION_SHARPNESS                                  , /**< Color image sharpness setting*/", "    RS2_OPTION_WHITE_BALANCE                              , /**< Controls white balance of color image. Setting any value will disable auto white balance*/", "    RS2_OPTION_ENABLE_AUTO_EXPOSURE                       , /**< Enable / disable color image auto-exposure*/", "    RS2_OPTION_ENABLE_AUTO_WHITE_BALANCE                  , /**< Enable / disable color image auto-white-balance*/", "    RS2_OPTION_VISUAL_PRESET                              , /**< Provide access to several recommend sets of option presets for the depth camera */", "    RS2_OPTION_LASER_POWER                                , /**< Power of the F200 / SR300 projector, with 0 meaning projector off*/", "    RS2_OPTION_ACCURACY                                   , /**< Set the number of patterns projected per frame. The higher the accuracy value the more patterns projected. Increasing the number of patterns help to achieve better accuracy. Note that this c", "    RS2_OPTION_MOTION_RANGE                               , /**< Motion vs. Range trade-off, with lower values allowing for better motion sensitivity and higher values allowing for better depth range*/", "    RS2_OPTION_FILTER_OPTION                              , /**< Set the filter to apply to each depth frame. Each one of the filter is optimized per the application requirements*/", "    RS2_OPTION_CONFIDENCE_THRESHOLD                       , /**< The confidence level threshold used by the Depth algorithm pipe to set whether a pixel will get a valid range or will be marked with invalid range*/", "    RS2_OPTION_EMITTER_ENABLED                            , /**< Laser Emitter enabled */", "    RS2_OPTION_FRAMES_QUEUE_SIZE                          , /**< Number of frames the user is allowed to keep per stream. Trying to hold-on to more frames will cause frame-drops.*/", "    RS2_OPTION_TOTAL_FRAME_DROPS                          , /**< Total number of detected frame drops from all streams */", "    RS2_OPTION_AUTO_EXPOSURE_MODE                         , /**< Auto-Exposure modes: Static, Anti-Flicker and Hybrid */", "    RS2_OPTION_POWER_LINE_FREQUENCY                       , /**< Power Line Frequency control for anti-flickering Off/50Hz/60Hz/Auto */", "    RS2_OPTION_ASIC_TEMPERATURE                           , /**< Current Asic Temperature */", "    RS2_OPTION_ERROR_POLLING_ENABLED                      , /**< disable error handling */", "    RS2_OPTION_PROJECTOR_TEMPERATURE                      , /**< Current Projector Temperature */", "    RS2_OPTION_OUTPUT_TRIGGER_ENABLED                     , /**< Enable / disable trigger to be outputed from the camera to any external device on every depth frame */", "    RS2_OPTION_MOTION_MODULE_TEMPERATURE                  , /**< Current Motion-Module Temperature */", "    RS2_OPTION_DEPTH_UNITS                                , /**< Number of meters represented by a single depth unit */", "    RS2_OPTION_ENABLE_MOTION_CORRECTION                   , /**< Enable/Disable automatic correction of the motion data */", "    RS2_OPTION_AUTO_EXPOSURE_PRIORITY                     , /**< Allows sensor to dynamically ajust the frame rate depending on lighting conditions */", "    RS2_OPTION_COUNT                                      , /**< Number of enumeration values. Not a valid input: intended to be used in for-loops. */"] ("RS Option")
        n37 = event-data() -> ("NewVal"=w92:bool)  [unwired: 1 in, 5 out]
        n38 = Boolean To (0,1)(Boolean=w92) -> (0, 1=w91:i16)
        n39 = call "rs3 set device option.vi"("value"=w91, "RS Option"=w93, "Sensor in"=w94) -> ()  [unwired: 6 in, 3 out]
      }
    }
    n40 = local read "stop"() -> (w61:bool)
  }
  n41 = while {
    tunnel: w38 -> [w121]
    tunnel: w30 -> [w131]
    tunnel: [w126] -> w37
    shift-right: [w100] -> _
    shift-left: sgl[][] [] ("2D Array Output") -> [w108]
    shift-right: [w102] -> _
    shift-left: u8[] [] ("Output Array") -> [w106]
    tunnel: w11 -> [w98]
    tunnel: w10 -> [w97]
    i -> [w130]
    stop <- "stop" stop-if-true
    # "8. Release Frames"
    # "7.  Display Frames, but for efficiency only update visible graphs"
    # "6. Interpret frames"
    # "5. Capture Frames"
    n42 = call "rs3 capture single 2.vi"("queue in"=w121, "error in (no error)"=w131) -> ("Capture Error"=→"Capture2 error":string, "frame out"=w129:u64, "width"=w101:i32, "Stream type"=w109:T8, "height"=w99:i32, "error out"=w122:errorcluster)  [unwired: 2 in, 6 out]
    n43 = call "rs3 capture single 2.vi"("queue in"=w121, "error in (no error)"=w122) -> ("Capture Error"=→"Capture1 Error":string, "frame out"=w119:u64, "width"=w111:i32, "Stream type"=w113:T8, "height"=w110:i32)  [unwired: 2 in, 7 out]
    n44 = call "rs3 get frame data2.vi"("frame in"=w129) -> ("error out"=w125:errorcluster, "image pointer out"=w128:u64, "Frame out"=w104:u64)  [unwired: 7 in, 1 out]
    n45 = call "rs3 get frame data2.vi"("error in (no error)"=w125, "frame in"=w119) -> ("error out"=w124:errorcluster, "image pointer out"=w112:u64, "Frame out"=w103:u64)  [unwired: 6 in, 1 out]
    n46 = case shown="\"Initialize\", Default" "Display tab" {
      tunnel: [TRUE ("Transpose") TRUE ("Transpose") FALSE ("Transpose") TRUE ("Transpose")] -> w95
      frame "Initialize", Default {
      }
      frame "Color + Depth" {
      }
      frame "PointCloud" {
      }
      frame "Errors" {
      }
    }
    n47 = case shown="\"IR Left\"" w109 {
      tunnel: [w208 w214 w222 w230] -> w115
      tunnel: w128 -> [_ w212 w225 w233]
      tunnel: w101 -> [_ w211 w224 w232]
      tunnel: w99 -> [_ w210 w223 w231]
      tunnel: w124 -> [w208 w215 w221 w229]
      tunnel: [w207 w216 w219 w227] -> w107
      tunnel: w108 -> [w207 _ w219 w227]
      tunnel: w106 -> [w206 w213 _ _]
      tunnel: [w206 w213 w220 w228] -> w105
      tunnel: w95 -> [_ w209 _ _]
      frame "Color (ext.)", Default {
      }
      frame "Depth" {
        w217 = u16 0 items=["Y16", "Y8"] ("Image format")
        # "Depth"
        n48 = call "rs3_MemCopyUINT16_3.vi"("Image format"=w217, "Transpose"=w209, "error in (no error)"=w215, "Depth Y"=w210, "Depth X"=w211, "Zimage pointer"=w212) -> ("error out"=w214:errorcluster, "2D Array Output"=w216:sgl[][])  [unwired: 2 in, 2 out]
      }
      frame "Color (left) " {
        w218 = enum16{"Monochrome", "RGB internal (RGB)"}."RGB internal (RGB)" ("Color format")
        # "Color"
        n49 = call "rs3_MemCopyRGB_IR2.vi"("Zimage pointer"=w225, "RGB  X, width"=w224, "RGB Y, height"=w223, "Color format"=w218, "error in (no error)"=w221) -> ("Output Array"=w220:u8[], "error out"=w222:errorcluster)  [unwired: 8 in, 1 out]
        n50 = local write "Color format"(w218) -> ()
      }
      frame "IR Left" {
        w226 = enum16{"Monochrome", "RGB internal (RGB)"}."Monochrome" ("Color format")
        # "Mono"
        n51 = call "rs3_MemCopyRGB_IR2.vi"("Zimage pointer"=w233, "RGB  X, width"=w232, "RGB Y, height"=w231, "Color format"=w226, "error in (no error)"=w229) -> ("Output Array"=w228:u8[], "error out"=w230:errorcluster)  [unwired: 8 in, 1 out]
        n52 = local write "Color format"(w226) -> ()
      }
    }
    n53 = case shown="\"IR Left\"" w113 {
      tunnel: [w182 w188 w198 w205] -> w114
      tunnel: w112 -> [_ w185 w197 w204]
      tunnel: w111 -> [_ w184 w196 w203]
      tunnel: w110 -> [_ w186 w195 w202]
      tunnel: w115 -> [w182 w189 _ _]
      tunnel: w107 -> [w181 _ w193 w200]
      tunnel: [w181 w190 w193 w200] -> w100
      tunnel: [w180 w191 w194 w201] -> w102
      tunnel: w105 -> [w180 w191 _ _]
      tunnel: w95 -> [_ w183 _ _]
      frame "Color (ext.)", Default {
      }
      frame "Depth" {
        w187 = u16 0 items=["Y16", "Y8"] ("Image format")
        # "Depth"
        n54 = call "rs3_MemCopyUINT16_3.vi"("Image format"=w187, "Transpose"=w183, "error in (no error)"=w189, "Depth Y"=w186, "Depth X"=w184, "Zimage pointer"=w185) -> ("error out"=w188:errorcluster, "2D Array Output"=w190:sgl[][])  [unwired: 2 in, 2 out]
      }
      frame "Color (left) " {
        w192 = enum16{"Monochrome", "RGB internal (RGB)"}."RGB internal (RGB)" ("Color format")
        # "Color"
        n55 = call "rs3_MemCopyRGB_IR2.vi"("Zimage pointer"=w197, "RGB  X, width"=w196, "RGB Y, height"=w195, "Color format"=w192) -> ("Output Array"=w194:u8[], "error out"=w198:errorcluster)  [unwired: 9 in, 1 out]
        n56 = local write "Color format"(w192) -> ()
      }
      frame "IR Left" {
        w199 = enum16{"Monochrome", "RGB internal (RGB)"}."Monochrome" ("Color format")
        # "Mono"
        n57 = call "rs3_MemCopyRGB_IR2.vi"("Zimage pointer"=w204, "RGB  X, width"=w203, "RGB Y, height"=w202, "Color format"=w199) -> ("Output Array"=w201:u8[], "error out"=w205:errorcluster)  [unwired: 9 in, 1 out]
        n58 = local write "Color format"(w199) -> ()
      }
    }
    n59 = case shown="\"PointCloud\"" "Display tab" {
      tunnel: w102 -> [_ w139 w159 _]
      tunnel: w101 -> [_ w141 w158 _]
      tunnel: w99 -> [_ w140 w157 _]
      tunnel: w100 -> [_ w138 w145 _]
      tunnel: w98 -> [_ _ w147 _]
      tunnel: w97 -> [_ _ w146 _]
      frame "Initialize", Default {
      }
      frame "Color + Depth" {
        (unwired) sgl[][] []  # Blank depthmap
        (unwired) picture bytes[33]  # Blank picture
        n60 = local read "Color format"() -> (w136:enum16{"Monochrome", "RGB internal (RGB)"})
        n61 = call "rs3_RGB_to_Picture5.vi"("RGB array"=w139, "Color format"=w136, "RGB  X, width"=w141, "RGB Y, height"=w140, "AWB"=FALSE, "White Balance"=FALSE) -> ("new picture"=→"RGB image":picture)  [unwired: 8 in, 1 out]
        "Depth map" <- w138
      }
      frame "PointCloud" {
        # "Convert color for 3D Picture format"
        # "Create x,y,z for PointCloud 3D Picture"
        n62 = for {
          tunnel: w145 -> [w162] mode=indexing
          tunnel: [w161] -> w151 mode=concatenating
          i -> [w160]
          n63 = for {
            tunnel: w162 -> [w179] mode=indexing
            tunnel: w160 -> [w178]
            tunnel: [w177] -> w161 mode=indexing
            i -> [w176]
            n64 = local read "ppx"() -> (w169:sgl)
            n65 = local read "ppy"() -> (w167:sgl)
            n66 = To Double Precision Float(number=w178) -> (double precision float=w166:dbl)
            n67 = To Double Precision Float(number=w176) -> (double precision float=w171:dbl)
            n68 = Subtract(x=w171, y=w169) -> (x-y=w170:dbl)
            n69 = Subtract(x=w166, y=w167) -> (x-y=w165:dbl)
            n70 = To Double Precision Float(number=w179) -> (double precision float=w164:dbl)
            n71 = Multiply(x=w164, y=w170) -> (x*y=w175:dbl)
            n72 = Multiply(x=w164, y=w165) -> (x*y=w172:dbl)
            n73 = local read "fx"() -> (w174:sgl)
            n74 = local read "fy"() -> (w168:sgl)
            n75 = Divide(x=w175, y=w174) -> (x/y=w173:dbl)
            n76 = Divide(x=w172, y=w168) -> (x/y=w163:dbl)
            n77 = Bundle(w173, w163, w164) -> (w177:cluster{dbl, dbl, dbl})  [unwired: 1 in]
          }
        }
        n78 = call "rs3_ExtractColor5.vi"("Manual \nWhite Balance"=FALSE ("White Balance"), "24bit Color Array"=w159, "Color format"="Color format", "Depth Y"=w157, "RGB  X"=w158, "RGB Y"=w157, "Depth X"=w158) -> ("Norm Mesh Color"=w150:T9)  [unwired: 8 in]
        n79 = call <vilib>:"Create Mesh.vi"() -> ("New Mesh Refnum"=w153:refnum<vi>)  [unwired: 10 in, 1 out]
        n80 = invoke class="SceneMesh" method="SetMeshParms"(reference=w153, "DrawMode"=T7."Points" ("Draw Mode"), "VertArray"=w151, "Indices"=w146, "ColorMode"=T6."Per Vertex" ("Color Binding Mode"), "ColorArray"=w150) -> (reference out=w154:refnum<vi>, error out=w155:errorcluster)  [unwired: 5 in, 9 out]
        n81 = invoke class="SceneObject" method="Set Drawable"(reference=w147, error in=w155, "Drawable"=w154) -> (reference out=→"3D Picture":refnum<vi>)  [unwired: 1 in, 3 out]
      }
      frame "Errors" {
      }
    }
    n82 = call "rs3 release frame.vi"("error in (no error)"=w114, "Frame"=w104) -> ("error out"=w127:errorcluster, "error"=w118:u64)  [unwired: 8 in]
    n83 = call "rs3 showError.vi"("error"=w118) -> ("Error summary"=→"release frame error":string)  [unwired: 6 in, 4 out]
    n84 = call "rs3 release frame.vi"("error in (no error)"=w127, "Frame"=w103) -> ("error out"=w126:errorcluster)  [unwired: 8 in, 1 out]
    "iteration" <- w130
  }
  n85 = flat-sequence {
    tunnel: [w238] -> w11
    tunnel: [w234] -> w10
    frame #0 {
      # "Cleate Point-Cloud Object"
      n86 = local read "height"() -> (w235:i32)
      n87 = local read "width"() -> (w236:i32)
      n88 = call <vilib>:"New Light.vi"("At Infinity"=TRUE) -> ("New Light Refnum"=w246:refnum<vi>)  [unwired: 2 in, 8 out]
      n89 = property class="SceneLight"(reference=w246, "Direction"=cluster{"X":sgl, "Y":sgl, "Z":sgl} {"X"=0.0, "Y"=0.0, "Z"=10000.0}, "Diffuse Color"=T12 {"Alpha"=1.0, "Blue"=1.0, "Green"=1.0, "Red"=1.0}, "atInfinity"=TRUE ("At Infinity"), "Light Number"=0, "Position"=T11 {"X"=10000.0, "Y"=0.0, "Z"=10000.0}, "Specular Color"=T10 {"Red"=1.0, "Green"=0.0, "Blue"=0.0, "Alpha"=0.0}) -> (reference out=w243:refnum<vi>)  [unwired: 1 in, 1 out]
      n90 = call-poly <vilib>:"Create Object.vi"("Name"="PointCloud Object") -> ("Scene:New Object"=w245:refnum<vi>)  [unwired: 9 in, 1 out]
      n91 = Multiply(x=w236, y=w235) -> (x*y=w237:i32)
      n92 = for {
        N: w237 -> [_]
        tunnel: [w250] -> w234 mode=indexing
        i -> [w250]
        # "indices"
      }
      n93 = invoke class="SceneObject" method="Light.Add Light"(reference=w245, "Light"=w243) -> (reference out=w238:refnum<vi>)  [unwired: 2 in, 3 out]
    }
  }
  n94 = call "rs3_close all2.vi"("rscontext"=w33, "queue in"=w38, "error in (no error)"=w37, "device_list"=w34, "Dev in"=w16, "Sensor in"=w27) -> ("Close Error"=→"Close Error":string)  [unwired: 4 in, 1 out]
